vi "UHR-Fleezers Control (host) - 12.7c.vi"() -> ()   [LabVIEW 2012] (continued)
        n2925 = xnode "Read/Write Control"("FPGA VI Reference In"=w4044, "error in"=w4043) -> ("FPGA VI Reference Out"=w4042:T20, "error out"=w4041:errorcluster, "APD 3 Gate Late Counter"=→"APD 3 Gate Late Counter":u8, "APD 3 Gate Relative Phase"=→"APD 3 Gate Relative Phase":i16)
      }
    }
    n2926 = Not Equal?(x=w3726, y="Calibration") -> (x != y?=w3685:bool)
    n2927 = case shown="True" w3685 {
      tunnel: w3724 -> [_ w4075]
      tunnel: w3723 -> [_ w4074]
      tunnel: w3722 -> [_ w4073]
      tunnel: w3719 -> [_ w4072]
      tunnel: w3659 -> [_ w4071]
      frame False {
      }
      frame True {
        n2928 = property on="Force" class="WFChart (strict)"("YScale.NameLbl.Text"=w4075) -> ()  [unwired: 2 in, 2 out]
        n2929 = property on="T2 X" class="DigNum (strict)"("Caption.Text"=w4073) -> ()  [unwired: 2 in, 2 out]
        n2930 = property on="T1 X" class="DigNum (strict)"("Caption.Text"=w4074) -> ()  [unwired: 2 in, 2 out]
        n2931 = property on="Mean" class="DigNum (strict)"("Caption.Text"=w4072) -> ()  [unwired: 2 in, 2 out]
        n2932 = property on="Difference" class="DigNum (strict)"("Caption.Text"=w4071) -> ()  [unwired: 2 in, 2 out]
      }
    }
    n2933 = Unbundle By Name(w3707) -> ("Y"=w3710:dbl[])
    n2934 = Unbundle By Name(w3704) -> ("Y"=w3713:dbl[])
    n2935 = Subtract(x=w3710, y=w3708) -> (x-y=w3711:dbl[])
    n2936 = Subtract(x=w3713, y=w3706) -> (x-y=w3712:dbl[])
    n2937 = Multiply(x=w3712, y="T2 alpha_x (nm/V)") -> (x*y=w3507:dbl[])
    n2938 = Multiply(x="T1 alpha_x (nm/V)", y=w3711) -> (x*y=w3508:dbl[])
    n2939 = Not(x="Trap Trig. Fl.") -> (.not. x?=w3544:bool)
    n2940 = Multiply(x=w3734, y=-1.0) -> (x*y=w3715:waveform(dbl))
    n2941 = Subtract(x=w3508, y=w3507) -> (x-y=w3703:dbl[])
    n2942 = Unbundle By Name(w3734) -> ("Y"=w3675:dbl[])
    n2943 = Unbundle By Name(w3735) -> ("Y"=w3509:dbl[])
    n2944 = Negate(x=w3703) -> (-x=w3505:dbl[])
    n2945 = Build Array(w3735, w3715) -> (→"Force":waveform(dbl)[])
    n2946 = Subtract(x=w3505, y="Offset (nm)") -> (x-y=w3673:dbl[])
    n2947 = call-poly <vilib>:"Mean.vi"("X"=w3675) -> ("mean"=w3511:dbl)  [unwired: 1 out]
    "T2 X" <- w3511
    n2948 = Negate(x=w3675) -> (-x=w3676:dbl[])
    n2949 = call-poly <vilib>:"Mean.vi"("X"=w3509) -> ("mean"=w3512:dbl)  [unwired: 1 out]
    "T1 X" <- w3512
    n2950 = Negate(x=w3511) -> (-x=w3510:dbl)
    n2951 = Bundle By Name(cluster=w3707, "Y"=w3673) -> (w3650:waveform(dbl))
    "Bead Separation" <- w3650
    n2952 = Add(x=w3509, y=w3676) -> (x+y=w3677:dbl[])
    n2953 = Add(x=w3512, y=w3510) -> (x+y=w3721:dbl)
    n2954 = Subtract(x=w3512, y=w3510) -> (x-y=→"Difference":dbl)
    n2955 = Divide(x=w3677, y=2.0) -> (x/y=→"Vec Mean of T1 T2":dbl[])
    n2956 = Divide(x=w3721, y=2.0) -> (x/y=w3679:dbl)
    "Mean" <- w3679
    n2957 = feedback-in #25("Trap Trig. Fl.") -> ()
    n2958 = feedback #25("Trap Trig. Fl.") -> (w3542:bool)
    n2959 = And(x=w3544, y=w3542) -> (x .and. y?=w3543:bool)
    n2960 = case "If have just turned off triggering" shown="True" w3543 {
      tunnel: w3525 -> [_ w3872]
      tunnel: w3524 -> [_ w3871]
      frame False {
      }
      frame True {
        w3870 = FALSE ("FPGA Trap Trig")
        n2961 = xnode "Read/Write Control"("FPGA VI Reference In"=w3872, "error in"=w3871, "FPGA Trap Trig"=w3870) -> ("FPGA VI Reference Out"=w3869:T20, "error out"=w3868:errorcluster)
        n2962 = xnode "Read/Write Control"("FPGA VI Reference In"=w3869, "error in"=w3868, "TTrig?"=w3870) -> ()  [unwired: 2 out]
        n2963 = local write "Initializing"(FALSE ("Initializing")) -> ()
        n2964 = local write "Triggered"(FALSE ("Triggered")) -> ()
        n2965 = local write "Waiting"(FALSE ("Waiting")) -> ()
      }
    }
    n2966 = Not(x=w3542) -> (.not. x?=w3555:bool)
    n2967 = And(x="Trap Trig. Fl.", y=w3555) -> (x .and. y?=w3552:bool)
    n2968 = local read "Tether"() -> (w3680:bool)
    n2969 = Or(x=w3552, y="Reinitialize") -> (x .or. y?=w3538:bool)
    n2970 = feedback #26(w3548) -> (w3553:string)
    n2971 = Select(t=w3548, s=w3552, f=w3553) -> (s? t:f=w3547:string)
    n2972 = Select(t=w3548, s="Reinitialize", f=w3547) -> (s? t:f=w3546:string)
    n2973 = feedback #27(0) -> (w3550:i32)
    n2974 = feedback #28(w3673) -> (w3672:dbl[])
    n2975 = Build Array (concatenate)(w3673, w3672) -> (w3506:dbl[])
    n2976 = case "For determining if there is a tether still" shown="True" w3680 {
      tunnel: w3679 -> [_ w3996]
      frame False {
      }
      frame True {
        n2977 = Greater?(x="Lost Tether Alarm Threshold (pN)", y=w3996) -> (0:w3994:bool)
        n2978 = case shown="True" w3994 {
          frame False {
          }
          frame True {
            w3997 = FALSE ("Value (Signaling)")
            n2979 = flat-sequence {
              frame #0 {
                # "stop only if saving"
                n2980 = local read "Saving..."() -> (w4009:bool)
                n2981 = And(x=w4009, y="TA Cancel Save?") -> (x .and. y?=w4008:bool)
                n2982 = local write "Stop Saving"(w4008) -> ()
              }
              frame #1 {
                n2983 = case shown="True" "TA Green Off?" {
                  frame False {
                  }
                  frame True {
                    w4012 = FALSE ("Fl. Triggered...")
                    n2984 = local write "Fl. Triggered..."(w4012) -> ()
                    n2985 = property on="Green Laser ON" class="Bool (strict)"("Val(Sgnl)"=w4012) -> ()  [unwired: 2 in, 2 out]
                  }
                }
              }
            }
            n2986 = local read "Time tether formed"() -> (w4003:timestamp)
            n2987 = Get Date/Time In Seconds() -> (seconds since 1Jan1904=w4004:timestamp)
            n2988 = Subtract(x=w4004, y=w4003) -> (x-y=w4002:dbl)
            n2989 = Number To Decimal String(number=w4002) -> (decimal integer string=w3999:string)  [unwired: 1 out]
            n2990 = local read "Messages"() -> (w4006:string)
            n2991 = call <vilib>:"Beep.vi"() -> ()  [unwired: 3 in, 9 out]
            n2992 = Concatenate Strings("Lost tether (" ("Message to add"), w3999, " s)." ("string")) -> (w4001:string)
            n2993 = local write "Tether"(FALSE ("Tether")) -> ()
            n2994 = call "Update messages.vi"("Message to add"=w4001, "Old message string"=w4006) -> ("New message string"=w4005:string)
            n2995 = local write "Messages"(w4005) -> ()
            n2996 = property on="Fl. Triggered..." class="Bool (strict)"("Val(Sgnl)"=w3997) -> ()  [unwired: 2 in, 2 out]
            n2997 = local write "Dip for Protein"(w3997) -> ()
            n2998 = property on="Trap Pos. FB ON" class="Bool (strict)"("Val(Sgnl)"=w3997) -> ()  [unwired: 2 in, 2 out]
            n2999 = property on="Trap Trig. Fl." class="Bool (strict)"("Val(Sgnl)"=w3997) -> ()  [unwired: 2 in, 2 out]
          }
        }
      }
    }
    n3000 = case "For triggering actions based on the trap position (e.g., turning the excitation laser on if trap under feedback moves so far)" shown="True" "Trap Trig. Fl." {
      tunnel: w3533 -> [_ w3885]
      tunnel: w3546 -> [_ w3884]
      tunnel: ["" ("t") w3883] -> w3554
      tunnel: w3538 -> [_ w3882]
      tunnel: [0 ("t") w3881] -> w3551
      tunnel: w3550 -> [_ w3880]
      tunnel: w3525 -> [_ w3879]
      tunnel: w3524 -> [_ w3878]
      frame False {
      }
      frame True {
        n3001 = case shown="\"Wait for trigger\"" w3884 {
          tunnel: w3885 -> [w3902 _ _ w3950]
          tunnel: [w3899 w3931 "" ("t") w3953] -> w3883
          tunnel: w3882 -> [_ _ _ w3941]
          tunnel: [w3898 w3928 0 ("t") w3942] -> w3881
          tunnel: w3880 -> [_ w3930 _ w3948]
          tunnel: w3879 -> [w3887 w3925 _ w3944]
          tunnel: w3878 -> [w3886 w3924 _ w3943]
          frame "Wait for trigger" {
            n3002 = local read "Trap Trig. (FPGA)"() -> (w3890:bool)
            n3003 = Subtract(x=w3902, y="Mean T1 Position\nto compare (nm)") -> (x-y=w3895:dbl[])
            n3004 = call <vilib>:"Std Deviation and Variance.vi"("X"=w3895) -> ("mean"=→"mean":dbl, "standard deviation"=→"standard\ndeviation":dbl)  [unwired: 1 in, 1 out]
            n3005 = Array Max & Min(array=w3895) -> (max value=→"max value":dbl, min value=→"min value":dbl)  [unwired: 2 out]
            n3006 = Greater?(x=w3895, y="Threshold (nm)") -> (0:w3905:bool[])
            n3007 = case shown="True" w3890 {
              tunnel: w3887 -> [_ w3911]
              tunnel: w3886 -> [_ w3910]
              tunnel: [FALSE ("TTrig?") w3909] -> w3893
              frame False {
              }
              frame True {
                n3008 = xnode "Read/Write Control"("FPGA VI Reference In"=w3911, "error in"=w3910) -> ("TTrig?"=w3909:bool)  [unwired: 2 out]
              }
            }
            n3009 = Or Array Elements(Boolean array=w3905) -> (logical OR=w3892:bool)
            n3010 = Select(t=w3893, s=w3890, f=w3892) -> (s? t:f=w3891:bool)
            n3011 = Not(x=w3890) -> (.not. x?=w3889:bool)
            n3012 = And(x=w3891, y=w3889) -> (x .and. y?=w3888:bool)
            n3013 = Select(t="Triggered", s=w3891, f="Wait for trigger") -> (s? t:f=w3899:string)
            n3014 = case shown="True" w3891 {
              tunnel: [0 0] -> w3898
              tunnel: w3887 -> [_ w3916]
              tunnel: w3886 -> [_ w3915]
              frame False {
                "Waiting" <- TRUE ("Waiting")
              }
              frame True {
                n3015 = xnode "Read/Write Control"("FPGA VI Reference In"=w3916, "error in"=w3915, "TTrig?"=FALSE) -> ()  [unwired: 2 out]
                n3016 = local read "Messages"() -> (w3919:string)
                n3017 = call <vilib>:"Beep.vi"() -> ()  [unwired: 12 in]
                n3018 = call "Update messages.vi"("Message to add"="Unwinding trigger.", "Old message string"=w3919) -> ("New message string"=w3920:string)
                n3019 = local write "Messages"(w3920) -> ()
                n3020 = local write "Waiting"(FALSE ("Waiting")) -> ()
                "Triggered" <- TRUE ("Triggered")
              }
            }
            n3021 = case "Only need to turn on laser if host triggered" shown="True" w3888 {
              frame False {
              }
              frame True {
                n3022 = property on="Green Laser ON" class="Bool (strict)"("Val(Sgnl)"=TRUE ("Value (Signaling)")) -> ()  [unwired: 2 in, 2 out]
              }
            }
          }
          frame "Triggered" {
            n3023 = local read "Trap Trig. (FPGA)"() -> (w3927:bool)
            n3024 = Increment(x=w3930) -> (x+1=w3928:i32)
            n3025 = Greater Or Equal?(x=w3928, y="Fl. ON time (n)") -> (x >= y?=w3926:bool)
            n3026 = Select(t="Wait for trigger", s=w3926, f="Triggered" ("t")) -> (s? t:f=w3931:string)
            n3027 = And(x=w3926, y=w3927) -> (x .and. y?=w3923:bool)
            n3028 = case shown="True" w3923 {
              tunnel: w3925 -> [_ w3935]
              tunnel: w3924 -> [_ w3934]
              frame False {
              }
              frame True {
                n3029 = xnode "Read/Write Control"("FPGA VI Reference In"=w3935, "error in"=w3934, "FPGA Trap Trig"=TRUE) -> ()  [unwired: 2 out]
              }
            }
            n3030 = case shown="True" w3926 {
              frame False {
              }
              frame True {
                w3937 = FALSE ("Value (Signaling)")
                n3031 = local write "Triggered"(w3937) -> ()
                n3032 = local write "Waiting"(TRUE ("Waiting")) -> ()
                n3033 = property on="Green Laser ON" class="Bool (strict)"("Val(Sgnl)"=w3937) -> ()  [unwired: 2 in, 2 out]
              }
            }
          }
          frame "Do nothing" {
          }
          frame "Initialize", Default {
            n3034 = Increment(x=w3948) -> (x+1=w3952:i32)
            n3035 = Select(t=1, s=w3941, f=w3952) -> (s? t:f=w3942:i32)
            n3036 = feedback #29(w3950) -> (w3956:dbl[])
            n3037 = Build Array (concatenate)(w3950, w3956) -> (w3949:dbl[])
            n3038 = Greater Or Equal?(x=w3942, y="Wait to get offset (n)") -> (x >= y?=w3945:bool)
            n3039 = Select(t=w3950, s=w3941, f=w3949) -> (s? t:f=w3951:dbl[])
            n3040 = feedback-in #29(w3951) -> ()
            n3041 = call-poly <vilib>:"Mean.vi"("X"=w3951) -> ("mean"=w3946:dbl)  [unwired: 1 out]
            n3042 = local write "Mean T1 Position\nto compare (nm)"(w3946) -> ()
            n3043 = case shown="True" w3941 {
              tunnel: w3944 -> [_ w3962]
              tunnel: w3943 -> [_ w3961]
              frame False {
              }
              frame True {
                w3958 = FALSE ("FPGA Trap Trig")
                n3044 = xnode "Read/Write Control"("FPGA VI Reference In"=w3962, "error in"=w3961, "FPGA Trap Trig"=w3958) -> ("FPGA VI Reference Out"=w3960:T20, "error out"=w3959:errorcluster)
                n3045 = xnode "Read/Write Control"("FPGA VI Reference In"=w3960, "error in"=w3959, "TTrig?"=w3958) -> ()  [unwired: 2 out]
              }
            }
            n3046 = Select(t="Wait for trigger", s=w3945, f="Initialize") -> (s? t:f=w3953:string)
            n3047 = case shown="True" w3945 {
              tunnel: w3946 -> [_ w3965]
              tunnel: w3944 -> [_ w3974]
              tunnel: w3943 -> [_ w3973]
              frame False {
                n3048 = local write "Waiting"(FALSE ("Waiting")) -> ()
                "Initializing" <- TRUE ("Initializing")
              }
              frame True {
                n3049 = local read "Threshold (nm)"() -> (w3977:dbl)
                n3050 = local read "AOM X Cal (nm/MHz)"() -> (w3976:dbl)
                n3051 = Add(x=w3965, y=w3977) -> (x+y=w3978:dbl)
                n3052 = Divide(x=w3978, y=w3976) -> (x/y=w3975:dbl)
                n3053 = call "IR AOM freq to word.vi"("Frequency In (MHz)"=w3975) -> ("Frequency Word Out (double)"=w3972:dbl)
                n3054 = local write "Initializing"(FALSE ("Initializing")) -> ()
                n3055 = local write "Waiting"(TRUE ("Waiting")) -> ()
                n3056 = To Quad Integer(1:w3972) -> (0:w3971:i64)
                n3057 = xnode "Read/Write Control"("FPGA VI Reference In"=w3974, "error in"=w3973, "FPGA TTrig Thresh"=w3971) -> ("FPGA VI Reference Out"=w3968:T20, "error out"=w3967:errorcluster)
                n3058 = xnode "Read/Write Control"("FPGA VI Reference In"=w3968, "error in"=w3967, "FPGA Trap Trig"=TRUE) -> ()  [unwired: 2 out]
              }
            }
          }
        }
      }
    }
    n3059 = feedback-in #26(w3554) -> ()
    n3060 = feedback-in #27(w3551) -> ()
    n3061 = Split 1D Array(array=w3506, index=w3568) -> (first subarray=w3669:dbl[])  [unwired: 1 out]
    n3062 = feedback-in #28(w3669) -> ()
    n3063 = call-poly <vilib>:"Mean.vi"("X"=w3669) -> ("mean"=w3668:dbl)  [unwired: 1 out]
    "Bead Mean (nm)" <- w3668
    n3064 = Subtract(x=w3669, y=w3668) -> (x-y=w3667:dbl[])
    n3065 = Square(x=w3667) -> (x^2=w3666:dbl[])
    n3066 = call-poly <vilib>:"Mean.vi"("X"=w3666) -> ("mean"=w3665:dbl)  [unwired: 1 out]
    n3067 = Square Root(x=w3665) -> (sqrt(x)=w3664:dbl)
    n3068 = Multiply(x=10.0, y=w3664) -> (x*y=→"RMS (Ang)":dbl)
    n3069 = xnode ("Read/Write Control")("FPGA VI Reference In"=w3701, "error in"=w3700) -> ("FPGA VI Reference Out"=w3536:T20, "error out"=w3535:errorcluster, "AI2 Y Sum Set 1"=w3799:i16, "AI2 Y Sum Set 2"=w3798:i16, "AI1 X Set 1"=w3600:fxp<+/-,16,1>, "AI1 X Set 2"=w3599:fxp<+/-,16,1>, "Trap Pos FB Int Signal"=→"Trap Pos FB Int Signal":fxp<+/-,24,9>, "Trap Pos FB Int-Norm Signal"=→"Trap Pos FB Int-Norm Signal":fxp<+/-,16,1>, "Trap Pos FB Action"=w3593:i64, "Scanning"=→"AOD Scanning":bool, "Scan I"=→"AOD Scan I":u64, "Scanning MCL"=w3801:bool, "Scan I (MCL)"=→"MCL Scan I":u64, "Green FB Sum"=w3738:i16, "Trap Pos FB Action"=w3523:i64, "TTrig Fin Thresh"=w3519:i64, "Red FB Intensity"=w3500:i16, "Blue Intensity"=w3495:i16)
    "MCL Scanning" <- w3801
    "Trap Pos FB Action" <- w3593
    n3070 = Divide(x=w3500, y=3276.7) -> (x/y=w3499:dbl)
    "Red laser intensity (V)" <- w3499
    n3071 = Divide(x=w3495, y=3276.7) -> (x/y=w3494:dbl)
    "Blue laser intensity (V)" <- w3494
    n3072 = Divide(x=w3738, y=3276.7) -> (x/y=w3498:dbl)
    "Green laser intensity (V)" <- w3498
    n3073 = local read "FB Trig Integrate"() -> (w3517:u32)
    n3074 = Divide(x=w3523, y=w3517) -> (x/y=w3516:dbl)
    "TTrig Sig (Int)" <- w3516
    n3075 = Bundle(w3498, w3499, w3494) -> (→"Fluorescence laser intensities plot":cluster{dbl, dbl, dbl})  [unwired: 1 in]
    n3076 = Divide(x=w3519, y=w3517) -> (x/y=w3514:dbl)
    "TTrig Fin Thresh (Int)" <- w3514
    n3077 = local read "AOM X Cal (nm/MHz)"() -> (w3522:dbl)
    n3078 = local read "AI2 (V)"() -> (w3800:cluster{"Set 1":dbl, "Set 2":dbl})
    n3079 = Bundle By Name(cluster=w3800, "Set 1"=w3799, "Set 2"=w3798) -> (w3796:cluster{"Set 1":dbl, "Set 2":dbl})
    n3080 = Divide(x=w3593, y=327.67) -> (x/y=→"Action (%)":dbl)
    n3081 = local read "Trap X (AI1)"() -> (w3613:T10)
    n3082 = call "IR AOM word double to freq.vi"("Frequency Word In (double)"=w3514) -> ("Frequency Out (MHz)"=w3513:dbl)
    n3083 = call "IR AOM word double to freq.vi"("Frequency Word In (double)"=w3516) -> ("Frequency Out (MHz)"=w3515:dbl)
    n3084 = Divide(x=w3796, y=3276.7) -> (x/y=w3795:cluster{"Set 1":dbl, "Set 2":dbl})
    n3085 = Multiply(x=w3515, y=w3522) -> (x*y=w3521:dbl)
    "TTrig Sig (nm)" <- w3521
    n3086 = Multiply(x=w3513, y=w3522) -> (x*y=w3520:dbl)
    "TTrig Fin Thresh (nm)" <- w3520
    n3087 = local write "AI2 (V)"(w3795) -> ()
    n3088 = Bundle(cluster=w3613, "Trap 1"=w3600, "Trap 2"=w3599) -> (→"Trap X (AI1)":T10)
    n3089 = Bundle(w3521, w3520) -> (→"TTrig":cluster{dbl, dbl})  [unwired: 1 in]
    n3090 = flat-sequence "To save data" {
      tunnel: [w4885] -> w3819
      tunnel: [w4886] -> w3818
      tunnel: w3769 -> [w4879]
      tunnel: w3541 -> [w4883]
      tunnel: ["Save Calibration"] -> w3792
      tunnel: w3789 -> [w4882]
      tunnel: [w4875] -> w3788
      tunnel: [w4872] -> w3787
      tunnel: [w4869] -> w3786
      tunnel: w3768 -> [w4871]
      tunnel: w3683 -> [w4865]
      tunnel: [w4865] -> w3682
      tunnel: ["Start Saving"] -> w3652
      tunnel: [w4859] -> w3581
      tunnel: [w4858] -> w3580
      tunnel: w3819 -> [w5133]
      tunnel: w3818 -> [w5132]
      tunnel: w3582 -> [w5131]
      tunnel: w3792 -> [w5130]
      tunnel: w3788 -> [w5128]
      tunnel: w3787 -> [w5127]
      tunnel: w3786 -> [w5126]
      tunnel: w3661 -> [w5125]
      tunnel: w3693 -> [w5124]
      tunnel: w3682 -> [w5123]
      tunnel: w3652 -> [w5122]
      tunnel: w3650 -> [w5121]
      tunnel: w3478 -> [w5120]
      tunnel: w3581 -> [w5119]
      tunnel: w3580 -> [w5118]
      tunnel: w3579 -> [w5117]
      tunnel: w3502 -> [w5116]
      frame #0 {
        n3091 = Or(x="Save N Sets", y="Start Saving") -> (x .or. y?=w4866:bool)
        n3092 = To Double Precision Float(number=w4882) -> (double precision float=w4876:dbl)
        n3093 = Build Array(w4866, "Save Calibration", w4879, w4871) -> (w4881:bool[])
        n3094 = Compound Arithmetic op=OR("Save Calibration", w4879, w4866, w4871) -> (w4884:bool)
        n3095 = Boolean Array To Number(Boolean array=w4881) -> (number=w4878:u32)
        n3096 = feedback #30(FALSE ("Save APD Data\nwith Trap Data")) -> (w4860:bool)
        n3097 = feedback #31(refnum<k0> refnum) -> (w4887:refnum<file>)
        n3098 = feedback #32(refnum<k0> refnum) -> (w4862:refnum<file>)
        n3099 = feedback #33(FALSE ("Save APD Data\nwith Trap Data")) -> (w4870:bool)
        n3100 = feedback #34(refnum<k0> refnum) -> (w4873:refnum<file>)
        n3101 = feedback #35(0) -> (w4889:i32)
        n3102 = feedback #36() -> (w4877:u32)  [unwired: 1 out]
        n3103 = case shown="True" w4884 {
          tunnel: [w4896 1] -> w4885
          tunnel: w4889 -> [w4898 _]
          tunnel: [w4897 w4929] -> w4886
          tunnel: w4887 -> [w4897 _]
          tunnel: w4883 -> [_ w4947]
          tunnel: w4876 -> [_ w4945]
          tunnel: w4878 -> [_ w4948]
          tunnel: [w4895 w4928] -> w4875
          tunnel: w4877 -> [w4895 _]
          tunnel: [w4894 w4926] -> w4872
          tunnel: w4873 -> [w4894 _]
          tunnel: [w4893 w4925] -> w4869
          tunnel: w4870 -> [w4893 _]
          tunnel: "Start Saving" -> [_ w4923]
          tunnel: w4865 -> [_ w4922]
          tunnel: [w4892 w4914] -> w4858
          tunnel: w4862 -> [w4892 _]
          tunnel: [w4891 w4913] -> w4859
          tunnel: w4860 -> [w4891 _]
          frame False {
            n3104 = Increment(x=w4898) -> (x+1=w4896:i32)
          }
          frame True {
            w4919 = FALSE ("Start Saving")
            w4924 = 9.0  # File Version
            w4931 = FALSE ("prepend array or string size? (T)")
            w4930 = T26."big-endian, network order" ("byte order (0:big-endian, network order)")
            n3105 = local read "BD 1 Frequency 1 (MHz)"() -> (w4944:dbl)
            n3106 = local read "BD 2 Frequency 1 (MHz)"() -> (w4943:dbl)
            n3107 = local read "BD 1 Frequency 2 (MHz)"() -> (w4942:dbl)
            n3108 = local read "BD 2 Frequency 2 (MHz)"() -> (w4941:dbl)
            n3109 = local read "BD 1 Frequency 3 (MHz)"() -> (w4940:dbl)
            n3110 = local read "BD 2 Frequency 3 (MHz)"() -> (w4939:dbl)
            n3111 = Array Size(array=w4922) -> (size(s)=w4921:i32)
            n3112 = To Double Precision Float(number=w4921) -> (double precision float=w4920:dbl)
            n3113 = local write "Save Calibration"(w4919) -> ()
            n3114 = local write "Start Saving"(w4919) -> ()
            n3115 = Build Array("Save APD Data\nwith Trap Data", "Save Trap Pos. Data") -> (w4916:bool[])
            n3116 = Boolean Array To Number(Boolean array=w4916) -> (number=w4915:u32)
            n3117 = Build Array(w4944, w4943, w4942, w4941, w4940, w4939) -> (w4938:dbl[])
            n3118 = case shown="1, Default" w4948 {
              tunnel: w4947 -> [w5020 w5040 w5056 w5094]
              tunnel: w4920 -> [w5025 w5047 w5076 w5113]
              tunnel: w4945 -> [w5024 w5046 w5075 w5112]
              tunnel: [w5021 w5042 w5067 w5104] -> w4936
              tunnel: [w5012 "Cal sets to save" w5057 w5095] -> w4928
              tunnel: w4938 -> [w5022 w5043 w5069 w5106]
              tunnel: "Save APD Data\nwith Trap Data" -> [w5019 _ w5053 w5092]
              tunnel: [w5019 w5034 w5053 w5092] -> w4925
              tunnel: w4924 -> [w5015 w5035 w5051 w5090]
              tunnel: w4923 -> [w5014 _ _ _]
              tunnel: [w5005 w5034 w5050 w5080] -> w4913
              tunnel: "Save Trap Pos. Data" -> [w5005 _ w5050 w5080]
              tunnel: w4915 -> [w5004 _ w5049 w5079]
              frame 1, Default {
                # "timeseries"
                n3119 = case shown="True" "Profile" {
                  tunnel: [w5028 w5032] -> w5009
                  tunnel: [w5028 w5031] -> w5008
                  tunnel: [w5028 w5030] -> w5007
                  tunnel: [w5028 w5029] -> w5006
                  frame False {
                    w5028 = 0.0 ("f")
                  }
                  frame True {
                    n3120 = local read "Current Position"() -> (w5033:cluster{dbl, dbl, dbl})
                    n3121 = local read "Y change (mm)"() -> (w5029:dbl)
                    n3122 = Unbundle(w5033) -> (w5032:dbl, w5031:dbl, w5030:dbl)
                  }
                }
                n3123 = local read "Save ave N"() -> (w5027:dbl)
                n3124 = Multiply(x=w5027, y=w5020) -> (x*y=w5026:dbl)
                n3125 = To Double Precision Float(number=w5004) -> (double precision float=w5018:dbl)
                n3126 = Build Array(w5015, w5020, w5026, w5025, w5024, 0.0 ("f")) -> (w5023:dbl[])
                n3127 = Build Array(w5018, w5009, w5008, w5007, w5006) -> (w5016:dbl[])
                n3128 = Select(t=u32 4000000000, s=w5014, f="N sets to save") -> (s? t:f=w5012:u32)
                n3129 = Build Array (concatenate)(w5023, w5022, w5016) -> (w5021:dbl[])
              }
              frame 2 {
                w5037 = 0.0 ("f")
                w5034 = FALSE ("Save APD Data\nwith Trap Data")
                # "calibration"
                n3130 = Boolean To (0,1)(Boolean=w5034) -> (0, 1=w5039:i16)
                n3131 = To Double Precision Float(number=w5039) -> (double precision float=w5038:dbl)
                n3132 = Build Array(w5038, w5037, w5037, w5037, w5037) -> (w5036:dbl[])
                n3133 = Build Array(w5035, w5040, w5040, w5047, w5046, 1.0 ("t")) -> (w5044:dbl[])
                n3134 = Build Array (concatenate)(w5044, w5043, w5036) -> (w5042:dbl[])
                "Calibrating Trap..." <- TRUE ("Calibrating...")
              }
              frame 4 {
                w5054 = 0.0 ("f")
                # "scan dir (x/y = 0/1)"
                # "cycles/step"
                # "n scans (f/b)"
                # "steps"
                # "freq. range"
                # "AOD raster scan"
                n3135 = local read "Number of F/B Scans (AOD)"() -> (w5061:u16)
                n3136 = local read "Cycles/step (AOD)"() -> (w5063:u64)
                n3137 = local read "Scan Range (MHz)"() -> (w5066:dbl)
                n3138 = local read "Scan steps (AOD)"() -> (w5065:u64)
                n3139 = local read "Scan BD"() -> (w5073:bool)
                n3140 = local read "Save ave N"() -> (w5078:dbl)
                n3141 = Boolean To (0,1)(Boolean=w5073) -> (0, 1=w5072:i16)
                n3142 = To Double Precision Float(number=w5061) -> (double precision float=w5060:dbl)
                n3143 = To Double Precision Float(number=w5065) -> (double precision float=w5064:dbl)
                n3144 = To Double Precision Float(number=w5063) -> (double precision float=w5062:dbl)
                n3145 = To Double Precision Float(number=w5072) -> (double precision float=w5071:dbl)
                n3146 = Multiply(x=w5078, y=w5056) -> (x*y=w5077:dbl)
                n3147 = To Double Precision Float(number=w5049) -> (double precision float=w5055:dbl)
                n3148 = Build Array(w5055, w5054, w5054, w5054, w5054) -> (w5052:dbl[])
                n3149 = local read "N sets should be saved"() -> (w5058:dbl)
                n3150 = Build Array(w5071, w5066, w5064, w5062, w5060) -> (w5068:dbl[])
                n3151 = Build Array(w5051, w5056, w5077, w5076, w5075, 2.0 ("t")) -> (w5070:dbl[])
                n3152 = Round Toward +Infinity(x=w5058) -> (ceil(x): smallest int >= x=w5059:dbl)
                n3153 = Build Array (concatenate)(w5070, w5069, w5052, w5068) -> (w5067:dbl[])
                n3154 = To Unsigned Long Integer(number=w5059) -> (unsigned 32bit integer=w5057:u32)
              }
              frame 8 {
                w5087 = 0.0 ("f")
                # "MCL raster scan"
                n3155 = local read "Number of scans (MCL)"() -> (w5082:u64)
                n3156 = local read "Scan lines (y)"() -> (w5081:u64)
                n3157 = local read "2D or 1D Scan"() -> (w5084:bool)
                n3158 = local read "Scan Range (V)\n(of steps)"() -> (w5103:dbl)
                n3159 = local read "Fast Scan Dir"() -> (w5110:bool)
                n3160 = local read "Cycles/step (MCL)"() -> (w5100:u64)
                n3161 = local read "Scan steps (MCL)"() -> (w5102:u64)
                n3162 = Select(t=w5081, s=w5084, f=w5082) -> (s? t:f=w5083:u64)
                n3163 = Boolean To (0,1)(Boolean=w5084) -> (0, 1=w5086:i16)
                n3164 = local read "Save ave N"() -> (w5115:dbl)
                n3165 = local read "Initial X"() -> (w5089:dbl)
                n3166 = local read "Initial Y"() -> (w5088:dbl)
                n3167 = To Double Precision Float(number=w5086) -> (double precision float=w5085:dbl)
                n3168 = Boolean To (0,1)(Boolean=w5110) -> (0, 1=w5109:i16)
                n3169 = To Double Precision Float(number=w5083) -> (double precision float=w5098:dbl)
                n3170 = To Double Precision Float(number=w5102) -> (double precision float=w5101:dbl)
                n3171 = To Double Precision Float(number=w5100) -> (double precision float=w5099:dbl)
                n3172 = To Double Precision Float(number=w5109) -> (double precision float=w5108:dbl)
                n3173 = Multiply(x=w5115, y=w5094) -> (x*y=w5114:dbl)
                n3174 = To Double Precision Float(number=w5079) -> (double precision float=w5093:dbl)
                n3175 = local read "N sets should be saved (MCL)"() -> (w5096:dbl)
                n3176 = Build Array(w5093, w5085, w5087, w5087, w5087) -> (w5091:dbl[])
                n3177 = Build Array(w5108, w5103, w5101, w5099, w5098, w5089, w5088) -> (w5105:dbl[])
                n3178 = Build Array(w5090, w5094, w5114, w5113, w5112, 3.0 ("t")) -> (w5107:dbl[])
                n3179 = Round Toward +Infinity(x=w5096) -> (ceil(x): smallest int >= x=w5097:dbl)
                n3180 = Build Array (concatenate)(w5107, w5106, w5091, w5105) -> (w5104:dbl[])
                n3181 = To Unsigned Long Integer(number=w5097) -> (unsigned 32bit integer=w5095:u32)
              }
            }
            n3182 = local read "Index"() -> (w4953:dbl)
            n3183 = call "Create new save file.vi"("Insert"="", "Ext"=".dat", "Index In"=w4953) -> ("Path Out"=w4909:path, "Index Out"=w4927:dbl)
            n3184 = local write "Save file name"(w4909) -> ()
            n3185 = local write "Index"(w4927) -> ()
            n3186 = local write "Save index"(w4927) -> ()
            n3187 = Array Size(array=w4936) -> (size(s)=w4937:i32)
            n3188 = Open/Create/Replace File(file path (use dialog)=w4909, operation (0:open)=T27."create", access (0:read/write)=enum16{"read/write", "read-only", "write-only"}."write-only") -> (refnum out=w4950:refnum<file>)  [unwired: 1 in, 4 out]
            n3189 = local write "Saving..."(TRUE ("Saving...")) -> ()
            n3190 = To Double Precision Float(number=w4937) -> (double precision float=w4935:dbl)
            n3191 = String Length(string="Comment (data description)") -> (length=w4934:i32)
            n3192 = To Double Precision Float(number=w4934) -> (double precision float=w4933:dbl)
            n3193 = Deny Access(7:w4950) -> (3:w4949:refnum<file>)  [unwired: 1 in, 2 out]
            n3194 = Build Array (concatenate)(w4935, w4936, w4933) -> (w4908:dbl[])
            n3195 = case "If fluorescence data to be saved" shown="True" w4925 {
              tunnel: w4909 -> [_ w5003]
              tunnel: [refnum<k0> refnum w4983] -> w4926
              frame False {
              }
              frame True {
                w4982 = 0.0
                n3196 = local read "APD Integration Time (s)"() -> (w4988:dbl)
                n3197 = local read "N APD Samp/step"() -> (w4981:dbl)
                n3198 = local read "Number of APDs"() -> (w4980:u8)
                n3199 = Path To String(path=w5003) -> (string=w5002:string)
                n3200 = String Length(string=w5002) -> (length=w5001:i32)
                n3201 = Subtract(x=w5001, y=4) -> (x-y=w4999:i32)
                n3202 = String Subset(string=w5002, length (rest)=w4999) -> (substring=w4998:string)  [unwired: 1 out]
                n3203 = Build Array(w4988, w4981, w4980, w4982, w4982, w4982, w4982, w4982) -> (w4985:dbl[])
                n3204 = Concatenate Strings(w4998, "_fl.dat" ("string")) -> (w4996:string)
                n3205 = Array Size(array=w4985) -> (size(s)=w4987:i32)
                n3206 = String To Path(string=w4996) -> (path=w4992:path)
                n3207 = Open/Create/Replace File(file path (use dialog)=w4992, operation (0:open)=T27."create", access (0:read/write)=enum16{"read/write", "read-only", "write-only"}."write-only") -> (refnum out=w4993:refnum<file>)  [unwired: 1 in, 4 out]
                n3208 = Deny Access(7:w4993) -> (3:w4989:refnum<file>)  [unwired: 1 in, 2 out]
                n3209 = To Double Precision Float(number=w4987) -> (double precision float=w4986:dbl)
                n3210 = Build Array (concatenate)(w4986, w4985) -> (w4984:dbl[])
                n3211 = Write to Binary File(file (use dialog)=w4989, data=w4984, 5:FALSE ("prepend array or string size? (T)"), 9:T26."big-endian, network order" ("byte order (0:big-endian, network order)")) -> (refnum out=w4983:refnum<file>)  [unwired: 1 in, 3 out]
              }
            }
            n3212 = case shown="True" w4913 {
              tunnel: w4909 -> [_ w4964]
              tunnel: [refnum<k0> refnum w4963] -> w4914
              frame False {
              }
              frame True {
                w4959 = 0.0 ("element")
                n3213 = Path To String(path=w4964) -> (string=w4978:string)
                n3214 = Build Array(w4959, w4959, w4959, w4959, w4959, w4959, w4959, w4959) -> (w4960:dbl[])
                n3215 = String Length(string=w4978) -> (length=w4977:i32)
                n3216 = Subtract(x=w4977, y=4) -> (x-y=w4975:i32)
                n3217 = Array Size(array=w4960) -> (size(s)=w4962:i32)
                n3218 = String Subset(string=w4978, length (rest)=w4975) -> (substring=w4974:string)  [unwired: 1 out]
                n3219 = To Double Precision Float(number=w4962) -> (double precision float=w4961:dbl)
                n3220 = Concatenate Strings(w4974, "_pos.dat" ("string")) -> (w4972:string)
                n3221 = Build Array (concatenate)(w4961, w4960) -> (w4958:dbl[])
                n3222 = String To Path(string=w4972) -> (path=w4968:path)
                n3223 = Open/Create/Replace File(file path (use dialog)=w4968, operation (0:open)=T27."create", access (0:read/write)=enum16{"read/write", "read-only", "write-only"}."write-only") -> (refnum out=w4969:refnum<file>)  [unwired: 1 in, 4 out]
                n3224 = Deny Access(7:w4969) -> (3:w4965:refnum<file>)  [unwired: 1 in, 2 out]
                n3225 = Write to Binary File(file (use dialog)=w4965, data=w4958, 5:FALSE ("prepend array or string size? (T)"), 9:T26."big-endian, network order" ("byte order (0:big-endian, network order)")) -> (refnum out=w4963:refnum<file>)  [unwired: 1 in, 3 out]
              }
            }
            n3226 = Write to Binary File(file (use dialog)=w4949, data=w4908, 5:w4931, 9:w4930) -> (refnum out=w4932:refnum<file>)  [unwired: 1 in, 3 out]
            n3227 = Write to Binary File(file (use dialog)=w4932, data="Comment (data description)", 5:w4931, 9:w4930) -> (refnum out=w4929:refnum<file>)  [unwired: 1 in, 3 out]
            n3228 = local read "connection reference"() -> (w4911:T17)
            n3229 = Bundle("Comment (data description)"="Comment (data description)", "Channel 1 Buffer"="Channel 1 Buffer", "Channel 2 Buffer"="Channel 2 Buffer", "Channel 3 Buffer"="Channel 3 Buffer", "Title"="Title", "DNA Construct"="DNA Construct", "Bead diameter"="Bead diameter", "Name"="Name") -> (w4899:T50)  [unwired: 1 in]
            n3230 = call "MattFileCreator-v9.vi"("Comments"=w4899, "Input Array"=w4908, "File path"=w4909, "table"="labview", "connection reference"=w4911) -> ("connection reference out"=w4910:T17)  [unwired: 5 in, 1 out]
            n3231 = local write "connection reference"(w4910) -> ()
          }
        }
        n3232 = feedback-in #30(w4859) -> ()
        n3233 = feedback-in #31(w4886) -> ()
        n3234 = feedback-in #32(w4858) -> ()
        n3235 = feedback-in #33(w4869) -> ()
        n3236 = feedback-in #34(w4872) -> ()
        n3237 = feedback-in #35(w4885) -> ()
        n3238 = feedback-in #36(w4875) -> ()
      }
      frame #1 {
        n3239 = local read "Saving..."() -> (w5129:bool)
        n3240 = case shown="True" w5129 {
          tunnel: w5133 -> [_ w5144]
          tunnel: w5132 -> [_ w5158]
          tunnel: w5131 -> [_ w5154]
          tunnel: w5130 -> [_ w5153]
          tunnel: w5128 -> [_ w5152]
          tunnel: w5127 -> [_ w5147]
          tunnel: w5126 -> [_ w5146]
          tunnel: w5125 -> [_ w5145]
          tunnel: w5124 -> [_ w5143]
          tunnel: w5123 -> [_ w5141]
          tunnel: w5122 -> [_ w5140]
          tunnel: w5121 -> [_ w5139]
          tunnel: w5120 -> [_ w5138]
          tunnel: w5119 -> [_ w5137]
          tunnel: w5118 -> [_ w5136]
          tunnel: w5117 -> [_ w5135]
          tunnel: w5116 -> [_ w5134]
          frame False {
          }
          frame True {
            n3241 = Multiply(x=w5144, y=w5143) -> (x*y=→"Time (s)":dbl)
            n3242 = Less Or Equal?(x=w5144, y=w5152) -> (x <= y?=w5156:bool)
            n3243 = Or(x="Stop Saving", y="Abort save 2") -> (x .or. y?=w5148:bool)
            n3244 = Not(x=w5148) -> (.not. x?=w5157:bool)
            n3245 = And(x=w5156, y=w5157) -> (x .and. y?=w5155:bool)
            n3246 = case shown="True" w5155 {
              tunnel: w5158 -> [w5165 w5256]
              tunnel: [0.0 w5259] -> w5151
              tunnel: w5144 -> [_ w5257]
              tunnel: w5152 -> [_ w5258]
              tunnel: w5154 -> [_ w5253]
              tunnel: w5153 -> [_ _]
              tunnel: w5147 -> [w5163 w5246]
              tunnel: w5146 -> [w5162 w5247]
              tunnel: w5145 -> [_ w5245]
              tunnel: w5141 -> [_ w5244]
              tunnel: w5140 -> [_ w5168]
              tunnel: w5139 -> [_ w5237]
              tunnel: w5138 -> [_ w5184]
              tunnel: w5137 -> [w5159 w5201]
              tunnel: w5136 -> [w5160 w5200]
              tunnel: w5135 -> [_ w5197]
              tunnel: w5134 -> [_ w5195]
              frame False {
                w5161 = FALSE
                n3247 = Close File(refnum=w5165) -> ()  [unwired: 1 in, 2 out]
                n3248 = case shown="True" w5162 {
                  tunnel: w5163 -> [_ w5167]
                  frame False {
                  }
                  frame True {
                    n3249 = Close File(refnum=w5167) -> ()  [unwired: 1 in, 2 out]
                  }
                }
                n3250 = case shown="True" w5159 {
                  tunnel: w5160 -> [_ w5166]
                  frame False {
                  }
                  frame True {
                    n3251 = Close File(refnum=w5166) -> ()  [unwired: 1 in, 2 out]
                  }
                }
                n3252 = local write "Raster Scanning..."(w5161) -> ()
                n3253 = local write "Calibrating Trap..."(w5161) -> ()
                n3254 = call <vilib>:"Beep.vi"() -> ()  [unwired: 3 in, 9 out]
                n3255 = local write "Stop Saving"(w5161) -> ()
                "Saving..." <- w5161
              }
              frame True {
                n3256 = local read "Calibrating Trap..."() -> (w5248:bool)
                n3257 = case "Write fl. data" shown="True" w5247 {
                  tunnel: w5246 -> [_ w5282]
                  tunnel: w5245 -> [_ w5281]
                  frame False {
                  }
                  frame True {
                    n3258 = Write to Binary File(file (use dialog)=w5282, data=w5281, 5:FALSE ("prepend array or string size? (T)"), 9:T26."big-endian, network order" ("byte order (0:big-endian, network order)")) -> ()  [unwired: 1 in, 4 out]
                  }
                }
                n3259 = Greater?(x="Save ave N", y=1.0) -> (0:w5251:bool)
                n3260 = Not(x=w5248) -> (.not. x?=w5250:bool)
                n3261 = And(x=w5250, y=w5251) -> (x .and. y?=w5198:bool)
                n3262 = case shown="True" w5198 {
                  tunnel: w5197 -> [w5262 w5273]
                  tunnel: [w5262 w5265] -> w5196
                  tunnel: "Save ave N" -> [_ w5266]
                  frame False {
                  }
                  frame True {
                    w5263 = 2 ("dimension size")
                    n3263 = Array Size(array=w5273) -> (size(s)=w5267:i32)
                    n3264 = Divide(x=w5267, y=w5263) -> (x/y=w5271:dbl)
                    n3265 = Reshape Array(w5273, w5271, w5263) -> (w5272:u64[][])
                    n3266 = Transpose 2D Array(2D array=w5272) -> (transposed array=w5270:u64[][])
                    n3267 = for {
                      tunnel: w5270 -> [w5275] mode=indexing
                      tunnel: [w5274] -> w5264 mode=indexing
                      tunnel: w5266 -> [w5276]
                      workers-P: _ -> [_]
                      n3268 = call "downsample 1D array - U64.vi"("Ave N"=w5276, "Array In"=w5275) -> ("Array Out"=w5274:u64[])  [unwired: 1 in]
                    }
                    n3269 = Transpose 2D Array(2D array=w5264) -> (transposed array=w5269:u64[][])
                    n3270 = Divide(x=w5267, y=w5266) -> (x/y=w5268:dbl)
                    n3271 = Reshape Array(w5269, w5268) -> (w5265:u64[])
                  }
                }
                n3272 = case shown="True" w5198 {
                  tunnel: w5253 -> [w5285 w5297]
                  tunnel: [w5285 w5289] -> w5249
                  tunnel: "Save ave N" -> [_ w5290]
                  tunnel: w5244 -> [_ w5288]
                  frame False {
                  }
                  frame True {
                    n3273 = Array Size(array=w5297) -> (size(s)=w5291:i32)
                    n3274 = Array Size(array=w5288) -> (size(s)=w5287:i32)
                    n3275 = Divide(x=w5291, y=w5287) -> (x/y=w5295:dbl)
                    n3276 = Reshape Array(w5297, w5295, w5287) -> (w5296:i16[][])
                    n3277 = Transpose 2D Array(2D array=w5296) -> (transposed array=w5294:i16[][])
                    n3278 = for {
                      tunnel: w5294 -> [w5300] mode=indexing
                      tunnel: [w5299] -> w5286 mode=indexing
                      tunnel: w5290 -> [w5298]
                      workers-P: _ -> [_]
                      n3279 = call "downsample 1D array - I16.vi"("Ave N"=w5298, "Array In"=w5300) -> ("Array Out"=w5299:i16[])  [unwired: 1 out]
                    }
                    n3280 = Transpose 2D Array(2D array=w5286) -> (transposed array=w5293:i16[][])
                    n3281 = Divide(x=w5291, y=w5290) -> (x/y=w5292:dbl)
                    n3282 = Reshape Array(w5293, w5292) -> (w5289:i16[])
                  }
                }
                n3283 = Index Array(array=w5184, index=2) -> (element=w5185:waveform(dbl))
                n3284 = Index Array(array=w5184, index=1) -> (element=w5218:waveform(dbl))
                n3285 = Index Array(array=w5184, index=0) -> (element=w5220:waveform(dbl))
                n3286 = Unbundle By Name(w5185) -> ("Y"=w5187:dbl[])
                n3287 = Unbundle By Name(w5218) -> ("Y"=w5222:dbl[])
                n3288 = Unbundle By Name(w5220) -> ("Y"=w5230:dbl[])
                n3289 = case "Write trap pos. data" shown="True" w5201 {
                  tunnel: w5200 -> [_ w5278]
                  tunnel: w5196 -> [_ w5277]
                  frame False {
                  }
                  frame True {
                    n3290 = Write to Binary File(file (use dialog)=w5278, data=w5277, 5:FALSE ("prepend array or string size? (T)"), 9:T26."big-endian, network order" ("byte order (0:big-endian, network order)")) -> ()  [unwired: 1 in, 4 out]
                  }
                }
                n3291 = Write to Binary File(file (use dialog)=w5256, data=w5249, 5:FALSE ("prepend array or string size? (T)"), 9:T26."big-endian, network order" ("byte order (0:big-endian, network order)")) -> ()  [unwired: 1 in, 4 out]
                n3292 = feedback #37(w5187) -> (w5188:dbl[])
                n3293 = Build Array (concatenate)(w5188, w5187) -> (w5183:dbl[])
                n3294 = Select(t=w5187, s=w5168, f=w5183) -> (s? t:f=w5173:dbl[])
                n3295 = feedback-in #37(w5173) -> ()
                n3296 = feedback #38(w5222) -> (w5224:dbl[])
                n3297 = Build Array (concatenate)(w5224, w5222) -> (w5223:dbl[])
                n3298 = Select(t=w5222, s=w5168, f=w5223) -> (s? t:f=w5212:dbl[])
                n3299 = feedback-in #38(w5212) -> ()
                n3300 = feedback #39(w5230) -> (w5243:dbl[])
                n3301 = Build Array (concatenate)(w5243, w5230) -> (w5242:dbl[])
                n3302 = Select(t=w5230, s=w5168, f=w5242) -> (s? t:f=w5217:dbl[])
                n3303 = feedback-in #39(w5217) -> ()
                n3304 = Divide(x=w5257, y=w5258) -> (x/y=w5260:dbl)
                n3305 = Multiply(x=w5260, y=100.0) -> (x*y=w5259:dbl)
                n3306 = Build Array(w5217, w5212, w5173) -> (→"Saved APD":dbl[][])
                n3307 = Array Size(array=w5217) -> (size(s)=w5235:i32)
                n3308 = Unbundle By Name(w5237) -> ("Y"=w5241:dbl[])
                n3309 = Subtract(x=w5235, y="N pts to average") -> (x-y=w5170:i32)
                n3310 = Multiply(x="N pts to average", y=u16 2) -> (x*y=w5213:u16)
                n3311 = Subtract(x=w5235, y=w5213) -> (x-y=w5171:i32)
                n3312 = feedback #40(w5241) -> (w5240:dbl[])
                n3313 = Build Array (concatenate)(w5240, w5241) -> (w5239:dbl[])
                n3314 = Select(t=w5241, s=w5168, f=w5239) -> (s? t:f=w5238:dbl[])
                "Trap Delta Graph" <- w5238
                n3315 = feedback-in #40(w5238) -> ()
                n3316 = Array Subset(array=w5217, index=w5170, length="N pts to average") -> (w5234:dbl[])
                n3317 = Array Subset(array=w5217, index=w5171, length="N pts to average") -> (w5233:dbl[])
                n3318 = Array Subset(array=w5212, index=w5170, length="N pts to average") -> (w5215:dbl[])
                n3319 = Array Subset(array=w5212, index=w5171, length="N pts to average") -> (w5214:dbl[])
                n3320 = Array Subset(array=w5173, index=w5170, length="N pts to average") -> (w5182:dbl[])
                n3321 = Array Subset(array=w5173, index=w5171, length="N pts to average") -> (w5181:dbl[])
                n3322 = Index Array(array=w5195, index=0) -> (element=w5193:waveform(dbl))
                n3323 = call-poly <vilib>:"Mean.vi"("X"=w5234) -> ("mean"=w5232:dbl)  [unwired: 1 out]
                n3324 = call-poly <vilib>:"Mean.vi"("X"=w5215) -> ("mean"=w5211:dbl)  [unwired: 1 out]
                n3325 = call-poly <vilib>:"Mean.vi"("X"=w5233) -> ("mean"=w5231:dbl)  [unwired: 1 out]
                n3326 = call-poly <vilib>:"Mean.vi"("X"=w5214) -> ("mean"=w5210:dbl)  [unwired: 1 out]
                n3327 = call-poly <vilib>:"Mean.vi"("X"=w5182) -> ("mean"=w5180:dbl)  [unwired: 1 out]
                n3328 = call-poly <vilib>:"Mean.vi"("X"=w5181) -> ("mean"=w5179:dbl)  [unwired: 1 out]
                n3329 = Unbundle By Name(w5193) -> ("Y"=w5191:dbl[])
                n3330 = Subtract(x=w5211, y=w5210) -> (x-y=w5202:dbl)
                "Delta Fl. 2" <- w5202
                n3331 = Subtract(x=w5180, y=w5179) -> (x-y=w5174:dbl)
                "Delta Fl. 3" <- w5174
                n3332 = Subtract(x=w5232, y=w5231) -> (x-y=w5229:dbl)
                "Delta Fl. 1" <- w5229
                n3333 = feedback #41(w5191) -> (w5190:dbl[])
                n3334 = Build Array (concatenate)(w5190, w5191) -> (w5192:dbl[])
                n3335 = Initialize Array(w5229, 1 ("dimension size")) -> (w5226:dbl[])
                n3336 = Initialize Array(w5202, 1 ("dimension size")) -> (w5207:dbl[])
                n3337 = Initialize Array(w5174, 1 ("dimension size")) -> (w5176:dbl[])
                n3338 = Select(t=w5191, s=w5168, f=w5192) -> (s? t:f=w5189:dbl[])
                "Saved trap pos" <- w5189
                n3339 = feedback-in #41(w5189) -> ()
                n3340 = feedback #42(w5226) -> (w5227:dbl[])
                n3341 = Build Array (concatenate)(w5227, w5226) -> (w5225:dbl[])
                n3342 = feedback #43(w5207) -> (w5208:dbl[])
                n3343 = feedback #44(w5176) -> (w5177:dbl[])
                n3344 = Build Array (concatenate)(w5208, w5207) -> (w5206:dbl[])
                n3345 = Build Array (concatenate)(w5177, w5176) -> (w5175:dbl[])
                n3346 = Select(t=w5226, s=w5168, f=w5225) -> (s? t:f=w5205:dbl[])
                n3347 = feedback-in #42(w5205) -> ()
                n3348 = Select(t=w5207, s=w5168, f=w5206) -> (s? t:f=w5204:dbl[])
                n3349 = feedback-in #43(w5204) -> ()
                n3350 = Select(t=w5176, s=w5168, f=w5175) -> (s? t:f=w5169:dbl[])
                n3351 = feedback-in #44(w5169) -> ()
                n3352 = Build Array(w5205, w5204, w5169) -> (→"Save APD Deriv":dbl[][])
              }
            }
            "Progress" <- w5151
            "Progress 2" <- w5151
          }
        }
      }
    }
    n3353 = local read "wait to reset values"() -> (w3803:bool)
    n3354 = Not(x=w3801) -> (.not. x?=w3804:bool)
    n3355 = And(x=w3804, y=w3803) -> (x .and. y?=w3805:bool)
    n3356 = case "Part of MCL raster scanning: returns to initial positions after scan done" shown="True" w3805 {
      tunnel: w3536 -> [w4679 w4686]
      tunnel: [w4679 w4685] -> w3807
      tunnel: w3535 -> [w4678 w4684]
      tunnel: [w4678 w4683] -> w3802
      frame False {
      }
      frame True {
        w4694 = 10.0 ("y")
        w4693 = 32767.0 ("y")
        # "to return scan values\nafter a synchronous \nAOM scan"
        n3357 = local read "AO2"() -> (w4687:dbl)
        n3358 = local read "AO1"() -> (w4688:dbl)
        n3359 = local write "wait to reset values"(FALSE ("wait to reset values")) -> ()
        n3360 = Multiply(x=w4688, y=w4693) -> (x*y=w4690:dbl)
        n3361 = Multiply(x=w4687, y=w4693) -> (x*y=w4692:dbl)
        n3362 = Divide(x=w4690, y=w4694) -> (x/y=w4689:dbl)
        n3363 = Divide(x=w4692, y=w4694) -> (x/y=w4691:dbl)
        n3364 = To Word Integer(number=w4689) -> (16bit integer=w4695:i16)
        n3365 = To Word Integer(number=w4691) -> (16bit integer=w4696:i16)
        n3366 = local read "Total Counts (ticks)"() -> (w4680:u16)
        n3367 = xnode "Read/Write Control"("FPGA VI Reference In"=w4686, "error in"=w4684, "AO1"=w4695, "AO2"=w4696, "MCL count"=w4680) -> ("FPGA VI Reference Out"=w4685:T20, "error out"=w4683:errorcluster)
        n3368 = local read "Scan Range (V)\n(of steps)"() -> (w4681:dbl)
        n3369 = property on="Scan Range (V)\n(of steps)" class="DigNum (strict)"("Val(Sgnl)"=w4681) -> ()  [unwired: 2 in, 2 out]
      }
    }
    n3370 = node-c288() -> ()  [unwired: 2 out]
  }
  n3371 = node-c288(w17) -> ()  [unwired: 1 out]
  n3372 = node-c288(w132) -> ()  [unwired: 1 out]
  n3373 = node-c288(w134) -> ()  [unwired: 1 out]
  n3374 = property on="Saved trap pos" class="WFGraph (strict)"("Visible"=FALSE) -> ()  [unwired: 2 in, 2 out]
  n3375 = property on="Trap Delta Graph" class="WFGraph (strict)"("Visible"=TRUE) -> ()  [unwired: 2 in, 2 out]
  n3376 = local write "Trap pos"(FALSE ("Trap pos")) -> ()
  n3377 = node-c288(w119) -> ()  [unwired: 1 out]
  n3378 = disable-structure shown="Disabled" {
    disable-tunnel: w123 -> [w5302 _]
    disable-tunnel: w122 -> [w5301 _]
    frame Disabled {
      n3379 = VISA Close(VISA resource name=w5302, error in (no error)=w5301) -> (error out=w5303:errorcluster)
      n3380 = call <vilib>:"Simple Error Handler.vi"("error in (no error)"=w5303) -> ()  [unwired: 1 in, 8 out]
    }
    frame Enabled {
    }
  }
  n3381 = node-c288(w130) -> ()  [unwired: 1 out]
  n3382 = node-c288(w205) -> ()  [unwired: 1 out]
  n3383 = flat-sequence {
    tunnel: w296 -> [w5307]
    tunnel: w298 -> [w5308]
    tunnel: [w5306] -> w277
    tunnel: [w5305] -> w276
    tunnel: w261 -> [_]
    tunnel: w213 -> [_]
    tunnel: w136 -> [_]
    tunnel: w277 -> [w5309]
    tunnel: w276 -> [w5310]
    frame #0 {
      w5304 = FALSE ("AI to FIFO")
      n3384 = xnode "Read/Write Control"("FPGA VI Reference In"=w5308, "error in"=w5307, "AI to FIFO"=w5304, "APD to FIFO"=w5304) -> ("FPGA VI Reference Out"=w5306:T20, "error out"=w5305:errorcluster)
    }
    frame #1 {
      n3385 = xnode "Close FPGA VI Reference"("FPGA VI Reference In"=w5309, "error in"=w5310) -> ("error out"=→"error out":errorcluster)
    }
  }
